vi "FlexMag - 24-03-2023.vi"() -> ()   [LabVIEW 2018] (continued)
            n4342 = Concatenate Strings("000000" ("string"), w7261) -> (w7255:string)
            n4343 = String Length(string=w7255) -> (length=w7257:i32)
            n4344 = Subtract(x=w7257, y=6) -> (x-y=w7259:i32)
            n4345 = String Subset(string=w7255, offset (0)=w7259) -> (substring=w7254:string)  [unwired: 1 out]
            n4346 = Concatenate Strings("#001R:" ("string"), w7254, "\r", "\n") -> (w7271:string)
            n4347 = VISA Write(VISA resource name=w7273, write buffer=w7271, error in (no error)=w7272) -> (VISA resource name out=w7246:refnum<visa-resource-name>, error out=w7245:errorcluster)  [unwired: 1 out]
            n4348 = stacked-sequence {
              tunnel: [w7279] -> w7253
              tunnel: w7246 -> [w7279]
              tunnel: [w7278] -> w7252
              tunnel: w7245 -> [w7278]
              frame #0 {
                n4349 = Wait (ms)(milliseconds to wait=u32 50) -> ()  [unwired: 1 out]
              }
            }
            n4350 = property class="Instr"(reference=w7253, error in=w7252) -> (reference out=w7249:refnum<visa-resource-name>, error out=w7251:errorcluster, "Serial Settings:Number of Bytes at Serial Port"=w7250:u32)
            n4351 = VISA Read(VISA resource name=w7249, byte count=w7250, error in (no error)=w7251) -> (VISA resource name out=w7248:refnum<visa-resource-name>, error out=w7247:errorcluster)  [unwired: 2 out]
            n4352 = local write "pcgv1 auto set position"(FALSE ("Pc_bv1_auto_set position")) -> ()
            n4353 = stacked-sequence {
              tunnel: [w7276] -> w7244
              tunnel: w7248 -> [w7276]
              tunnel: [w7275] -> w7243
              tunnel: w7247 -> [w7275]
              frame #0 {
                n4354 = Wait (ms)(milliseconds to wait=u32 50) -> ()  [unwired: 1 out]
              }
            }
          }
          frame 4 {
            n4355 = Multiply(x="pcgv1 set pressure value mbar", y=u16 750) -> (x*y=w7280:dbl)
            "pcgv1 setted pressure value torr" <- w7280
            n4356 = Multiply(x=w7280, y=10000.0) -> (x*y=w7301:dbl)
            n4357 = Number To Decimal String(number=w7301) -> (decimal integer string=w7295:string)  [unwired: 1 out]
            n4358 = Concatenate Strings("00000000" ("string"), w7295) -> (w7297:string)
            n4359 = String Length(string=w7297) -> (length=w7298:i32)
            n4360 = Subtract(x=w7298, y=8) -> (x-y=w7300:i32)
            n4361 = String Subset(string=w7297, offset (0)=w7300) -> (substring=w7294:string)  [unwired: 1 out]
            n4362 = Concatenate Strings("#001S:" ("string"), w7294, "\r", "\n") -> (w7302:string)
            n4363 = VISA Write(VISA resource name=w7309, write buffer=w7302, error in (no error)=w7308) -> (VISA resource name out=w7286:refnum<visa-resource-name>, error out=w7285:errorcluster)  [unwired: 1 out]
            n4364 = stacked-sequence {
              tunnel: [w7315] -> w7293
              tunnel: w7286 -> [w7315]
              tunnel: [w7314] -> w7292
              tunnel: w7285 -> [w7314]
              frame #0 {
                n4365 = Wait (ms)(milliseconds to wait=u32 50) -> ()  [unwired: 1 out]
              }
            }
            n4366 = property class="Instr"(reference=w7293, error in=w7292) -> (reference out=w7289:refnum<visa-resource-name>, error out=w7291:errorcluster, "Serial Settings:Number of Bytes at Serial Port"=w7290:u32)
            n4367 = VISA Read(VISA resource name=w7289, byte count=w7290, error in (no error)=w7291) -> (VISA resource name out=w7288:refnum<visa-resource-name>, error out=w7287:errorcluster)  [unwired: 2 out]
            n4368 = stacked-sequence {
              tunnel: [w7312] -> w7284
              tunnel: w7288 -> [w7312]
              tunnel: [w7311] -> w7283
              tunnel: w7287 -> [w7311]
              frame #0 {
                n4369 = Wait (ms)(milliseconds to wait=u32 50) -> ()  [unwired: 1 out]
              }
            }
            n4370 = local write "pcgv1 auto set pressure"(FALSE ("Pc_bv1_auto_set_pressure")) -> ()
          }
          frame 5 {
            n4371 = local write "Baratron1 auto set zero"(FALSE ("Pc_bv1_auto_baratron_set_zero")) -> ()
            n4372 = Concatenate Strings("#001Z:" ("string"), "\r", "\n") -> (w7329:string)
            n4373 = VISA Write(VISA resource name=w7333, write buffer=w7329, error in (no error)=w7332) -> (VISA resource name out=w7319:refnum<visa-resource-name>, error out=w7318:errorcluster)  [unwired: 1 out]
            n4374 = stacked-sequence {
              tunnel: [w7339] -> w7326
              tunnel: w7319 -> [w7339]
              tunnel: [w7338] -> w7325
              tunnel: w7318 -> [w7338]
              frame #0 {
                n4375 = Wait (ms)(milliseconds to wait=u32 50) -> ()  [unwired: 1 out]
              }
            }
            n4376 = property class="Instr"(reference=w7326, error in=w7325) -> (reference out=w7322:refnum<visa-resource-name>, error out=w7324:errorcluster, "Serial Settings:Number of Bytes at Serial Port"=w7323:u32)
            n4377 = VISA Read(VISA resource name=w7322, byte count=w7323, error in (no error)=w7324) -> (VISA resource name out=w7321:refnum<visa-resource-name>, error out=w7320:errorcluster)  [unwired: 2 out]
            n4378 = stacked-sequence {
              tunnel: [w7336] -> w7317
              tunnel: w7321 -> [w7336]
              tunnel: [w7335] -> w7316
              tunnel: w7320 -> [w7335]
              frame #0 {
                n4379 = Wait (ms)(milliseconds to wait=u32 50) -> ()  [unwired: 1 out]
              }
            }
          }
          frame 6 {
            n4380 = Concatenate Strings("#001L:" ("string"), "Learn value", "\r", "\n") -> (w7353:string)
            n4381 = VISA Write(VISA resource name=w7357, write buffer=w7353, error in (no error)=w7356) -> (VISA resource name out=w7343:refnum<visa-resource-name>, error out=w7342:errorcluster)  [unwired: 1 out]
            n4382 = stacked-sequence {
              tunnel: [w7363] -> w7350
              tunnel: w7343 -> [w7363]
              tunnel: [w7362] -> w7349
              tunnel: w7342 -> [w7362]
              frame #0 {
                n4383 = Wait (ms)(milliseconds to wait=u32 50) -> ()  [unwired: 1 out]
              }
            }
            n4384 = property class="Instr"(reference=w7350, error in=w7349) -> (reference out=w7346:refnum<visa-resource-name>, error out=w7348:errorcluster, "Serial Settings:Number of Bytes at Serial Port"=w7347:u32)
            n4385 = VISA Read(VISA resource name=w7346, byte count=w7347, error in (no error)=w7348) -> (VISA resource name out=w7345:refnum<visa-resource-name>, error out=w7344:errorcluster)  [unwired: 2 out]
            n4386 = stacked-sequence {
              tunnel: [w7360] -> w7341
              tunnel: w7345 -> [w7360]
              tunnel: [w7359] -> w7340
              tunnel: w7344 -> [w7359]
              frame #0 {
                n4387 = Wait (ms)(milliseconds to wait=u32 50) -> ()  [unwired: 1 out]
              }
            }
          }
        }
      }
      frame #1 {
        n4388 = Or(x="pcgv2 set position gui", y="pcgv2 auto set position") -> (x .or. y?=w7386:bool)
        n4389 = Or(x="pcgv2 set pressure gui", y="pcgv2 auto set pressure") -> (x .or. y?=w7385:bool)
        n4390 = Compound Arithmetic op=OR("pcgv2 open gui 2", "pcgv2 open gui 1", "pcgv2 open gui", "pcgv2 auto open") -> (w7371:bool)
        n4391 = Compound Arithmetic op=OR("pcgv2 close gui 2", "pcgv2 close gui 1", "pcgv2 auto close", "pcgv2 close gui") -> (w7370:bool)
        n4392 = Or(x="Baratron2 set zero gui", y="Baratron2 auto set zero") -> (x .or. y?=w7384:bool)
        n4393 = Build Array(FALSE, w7371, w7370, w7386, w7385, w7384) -> (w7388:bool[])
        n4394 = Boolean Array To Number(Boolean array=w7388) -> (number=w7390:u32)
        n4395 = Mantissa & Exponent(0:w7390) -> (2:w7389:dbl)  [unwired: 1 out]
        n4396 = case shown="0, Default" w7389 {
          tunnel: [w7394 w7463 w7486 w7509 w7549 w7583] -> w7368
          tunnel: [w7393 w7464 w7485 w7510 w7550 w7582] -> w7367
          tunnel: w7369 -> [w7392 w7473 w7497 w7521 w7561 w7594]
          tunnel: w7366 -> [w7391 w7472 w7496 w7520 w7560 w7593]
          frame 0, Default {
            n4397 = stacked-sequence {
              seq-local: [_ w7399 _ _ _] -> [_ _ _ w7436 _]
              seq-local: [_ w7398 _ _ _] -> [_ _ _ w7435 _]
              tunnel: [_ _ _ w7438 _] -> w7394
              tunnel: [_ _ _ w7437 _] -> w7393
              tunnel: w7392 -> [_ w7397 _ _ _]
              tunnel: w7391 -> [_ w7396 _ _ _]
              frame #0 {
                n4398 = Wait (ms)(milliseconds to wait=u32 50) -> ()  [unwired: 1 out]
              }
              frame #1 {
                n4399 = Concatenate Strings("#002A:" ("string"), "\r", "\n") -> (w7415:string)
                n4400 = VISA Write(VISA resource name=w7397, write buffer=w7415, error in (no error)=w7396) -> (VISA resource name out=w7413:refnum<visa-resource-name>, error out=w7412:errorcluster)  [unwired: 1 out]
                n4401 = stacked-sequence {
                  tunnel: [w7420] -> w7411
                  tunnel: w7413 -> [w7420]
                  tunnel: [w7419] -> w7410
                  tunnel: w7412 -> [w7419]
                  frame #0 {
                    n4402 = Wait (ms)(milliseconds to wait=u32 50) -> ()  [unwired: 1 out]
                  }
                }
                n4403 = property class="Instr"(reference=w7411, error in=w7410) -> (reference out=w7407:refnum<visa-resource-name>, error out=w7409:errorcluster, "Serial Settings:Number of Bytes at Serial Port"=w7408:u32)
                n4404 = VISA Read(VISA resource name=w7407, byte count=w7408, error in (no error)=w7409) -> (VISA resource name out=w7399:refnum<visa-resource-name>, read buffer=w7401:string, error out=w7398:errorcluster)  [unwired: 1 out]
                n4405 = Match Pattern(string=w7401, regular expression="#002A:") -> (after substring=w7405:string)  [unwired: 1 in, 3 out]
                n4406 = String Subset(string=w7405, offset (0)=0, length (rest)=3 ("length (rest)")) -> (substring=w7402:string)
                n4407 = Decimal String To Number(string=w7402) -> (number=→"pcgv2 position":i32)  [unwired: 2 in, 1 out]
              }
              frame #2 {
                n4408 = Wait (ms)(milliseconds to wait=u32 50) -> ()  [unwired: 1 out]
              }
              frame #3 {
                n4409 = Concatenate Strings("#002P:" ("string"), "\r", "\n") -> (w7452:string)
                n4410 = VISA Write(VISA resource name=w7436, write buffer=w7452, error in (no error)=w7435) -> (VISA resource name out=w7450:refnum<visa-resource-name>, error out=w7449:errorcluster)  [unwired: 1 out]
                n4411 = stacked-sequence {
                  tunnel: [w7459] -> w7448
                  tunnel: w7450 -> [w7459]
                  tunnel: [w7458] -> w7447
                  tunnel: w7449 -> [w7458]
                  frame #0 {
                    n4412 = Wait (ms)(milliseconds to wait=u32 50) -> ()  [unwired: 1 out]
                  }
                }
                n4413 = property class="Instr"(reference=w7448, error in=w7447) -> (reference out=w7444:refnum<visa-resource-name>, error out=w7446:errorcluster, "Serial Settings:Number of Bytes at Serial Port"=w7445:u32)
                n4414 = VISA Read(VISA resource name=w7444, byte count=w7445, error in (no error)=w7446) -> (VISA resource name out=w7438:refnum<visa-resource-name>, read buffer=w7439:string, error out=w7437:errorcluster)  [unwired: 1 out]
                n4415 = Match Pattern(string=w7439, regular expression="#002P:") -> (after substring=w7427:string)  [unwired: 1 in, 3 out]
                n4416 = String Subset(string=w7427, offset (0)=0, length (rest)=1 ("length (rest)")) -> (substring=w7430:string)
                n4417 = String Subset(string=w7427, offset (0)=2, length (rest)=4 ("length (rest)")) -> (substring=w7440:string)
                n4418 = Equal?(x=w7430, y="-") -> (x = y?=w7428:bool)
                n4419 = Decimal String To Number(string=w7440) -> (number=w7434:i32)  [unwired: 2 in, 1 out]
                n4420 = case shown="True" w7428 {
                  frame False {
                  }
                  frame True {
                    w7455 = u16 0 ("Ch2_baratron_pressure_mbar")
                    w7456 = 0 ("Pressure 2")
                    n4421 = local write "Pressure 2_gui"(w7456) -> ()
                    n4422 = local write "Pressure 2_gui 2"(w7456) -> ()
                    n4423 = local write "Pressure 2"(w7456) -> ()
                    n4424 = local write "Ch2_baratron_pressure_mbar 2"(w7455) -> ()
                    n4425 = local write "Ch2_baratron_pressure_mbar"(w7455) -> ()
                    n4426 = local write "Ch2_baratron_pressure_mbar 3"(w7455) -> ()
                  }
                }
                n4427 = Divide(x=w7434, y=100) -> (x/y=w7425:dbl)
                "Pressure 2" <- w7425
                "Pressure 2_gui" <- w7425
                "Pressure 2_gui 2" <- w7425
                n4428 = Multiply(x=w7425, y=0.00133) -> (x*y=w7424:dbl)
                "Ch2_baratron_pressure_mbar" <- w7424
                "Ch2_baratron_pressure_mbar 2" <- w7424
                "Ch2_baratron_pressure_mbar 3" <- w7424
                n4429 = Number To Exponential String(number=w7424, precision (6)=i16 3) -> (E-format string=→"CH2 CH BG":string)  [unwired: 2 in]
              }
              frame #4 {
                n4430 = Wait (ms)(milliseconds to wait=u32 50) -> ()  [unwired: 1 out]
              }
            }
          }
          frame 1 {
            n4431 = Concatenate Strings("#002O:" ("string"), "\r", "\n") -> (w7476:string)
            n4432 = VISA Write(VISA resource name=w7473, write buffer=w7476, error in (no error)=w7472) -> (VISA resource name out=w7461:refnum<visa-resource-name>, error out=w7462:errorcluster)  [unwired: 1 out]
            n4433 = stacked-sequence {
              tunnel: [w7484] -> w7471
              tunnel: w7461 -> [w7484]
              tunnel: [w7483] -> w7470
              tunnel: w7462 -> [w7483]
              frame #0 {
                n4434 = Wait (ms)(milliseconds to wait=u32 50) -> ()  [unwired: 1 out]
              }
            }
            n4435 = local write "pcgv2 auto open"(FALSE ("Pc_bv2_auto_open")) -> ()
            n4436 = property class="Instr"(reference=w7471, error in=w7470) -> (reference out=w7467:refnum<visa-resource-name>, error out=w7469:errorcluster, "Serial Settings:Number of Bytes at Serial Port"=w7468:u32)
            n4437 = VISA Read(VISA resource name=w7467, byte count=w7468, error in (no error)=w7469) -> (VISA resource name out=w7466:refnum<visa-resource-name>, error out=w7465:errorcluster)  [unwired: 2 out]
            n4438 = stacked-sequence {
              tunnel: [w7481] -> w7463
              tunnel: w7466 -> [w7481]
              tunnel: [w7480] -> w7464
              tunnel: w7465 -> [w7480]
              frame #0 {
                n4439 = Wait (ms)(milliseconds to wait=u32 50) -> ()  [unwired: 1 out]
              }
            }
          }
          frame 2 {
            n4440 = Concatenate Strings("#002C:" ("string"), "\r", "\n") -> (w7500:string)
            n4441 = VISA Write(VISA resource name=w7497, write buffer=w7500, error in (no error)=w7496) -> (VISA resource name out=w7488:refnum<visa-resource-name>, error out=w7487:errorcluster)  [unwired: 1 out]
            n4442 = local write "pcgv2 auto close"(FALSE ("Pc_bv2_auto_close")) -> ()
            n4443 = stacked-sequence {
              tunnel: [w7508] -> w7495
              tunnel: w7488 -> [w7508]
              tunnel: [w7507] -> w7494
              tunnel: w7487 -> [w7507]
              frame #0 {
                n4444 = Wait (ms)(milliseconds to wait=u32 50) -> ()  [unwired: 1 out]
              }
            }
            n4445 = property class="Instr"(reference=w7495, error in=w7494) -> (reference out=w7491:refnum<visa-resource-name>, error out=w7493:errorcluster, "Serial Settings:Number of Bytes at Serial Port"=w7492:u32)
            n4446 = VISA Read(VISA resource name=w7491, byte count=w7492, error in (no error)=w7493) -> (VISA resource name out=w7490:refnum<visa-resource-name>, error out=w7489:errorcluster)  [unwired: 2 out]
            n4447 = stacked-sequence {
              tunnel: [w7505] -> w7486
              tunnel: w7490 -> [w7505]
              tunnel: [w7504] -> w7485
              tunnel: w7489 -> [w7504]
              frame #0 {
                n4448 = Wait (ms)(milliseconds to wait=u32 50) -> ()  [unwired: 1 out]
              }
            }
          }
          frame 3 {
            n4449 = In Range and Coerce(upper limit=100.0, x="pcgv2 set position value", lower limit=0.0) -> (coerced(x)=w7523:dbl)  [unwired: 1 out]
            n4450 = Multiply(x=w7523, y=1000.0) -> (x*y=w7530:dbl)
            n4451 = Number To Decimal String(number=w7530) -> (decimal integer string=w7532:string)  [unwired: 1 out]
            n4452 = Concatenate Strings("000000" ("string"), w7532) -> (w7534:string)
            n4453 = String Length(string=w7534) -> (length=w7535:i32)
            n4454 = Subtract(x=w7535, y=6) -> (x-y=w7537:i32)
            n4455 = String Subset(string=w7534, offset (0)=w7537) -> (substring=w7527:string)  [unwired: 1 out]
            n4456 = Concatenate Strings("#002R:" ("string"), w7527, "\r", "\n") -> (w7539:string)
            n4457 = VISA Write(VISA resource name=w7521, write buffer=w7539, error in (no error)=w7520) -> (VISA resource name out=w7513:refnum<visa-resource-name>, error out=w7512:errorcluster)  [unwired: 1 out]
            n4458 = stacked-sequence {
              tunnel: [w7544] -> w7514
              tunnel: w7513 -> [w7544]
              tunnel: [w7543] -> w7511
              tunnel: w7512 -> [w7543]
              frame #0 {
                n4459 = Wait (ms)(milliseconds to wait=u32 50) -> ()  [unwired: 1 out]
              }
            }
            n4460 = property class="Instr"(reference=w7514, error in=w7511) -> (reference out=w7517:refnum<visa-resource-name>, error out=w7519:errorcluster, "Serial Settings:Number of Bytes at Serial Port"=w7518:u32)
            n4461 = VISA Read(VISA resource name=w7517, byte count=w7518, error in (no error)=w7519) -> (VISA resource name out=w7516:refnum<visa-resource-name>, error out=w7515:errorcluster)  [unwired: 2 out]
            n4462 = local write "pcgv2 auto set position"(FALSE ("Pc_bv2_auto_set position")) -> ()
            n4463 = stacked-sequence {
              tunnel: [w7542] -> w7509
              tunnel: w7516 -> [w7542]
              tunnel: [w7541] -> w7510
              tunnel: w7515 -> [w7541]
              frame #0 {
                n4464 = Wait (ms)(milliseconds to wait=u32 50) -> ()  [unwired: 1 out]
              }
            }
          }
          frame 4 {
            n4465 = Multiply(x="pcgv2 set pressure value mbar", y=u16 750) -> (x*y=w7546:dbl)
            "pcgv2 setted pressure value torr" <- w7546
            n4466 = Multiply(x=w7546, y=10000.0) -> (x*y=w7566:dbl)
            n4467 = Number To Decimal String(number=w7566) -> (decimal integer string=w7568:string)  [unwired: 1 out]
            n4468 = Concatenate Strings("00000000" ("string"), w7568) -> (w7570:string)
            n4469 = String Length(string=w7570) -> (length=w7571:i32)
            n4470 = Subtract(x=w7571, y=8) -> (x-y=w7573:i32)
            n4471 = String Subset(string=w7570, offset (0)=w7573) -> (substring=w7563:string)  [unwired: 1 out]
            n4472 = Concatenate Strings("#002S:" ("string"), w7563, "\r", "\n") -> (w7575:string)
            n4473 = VISA Write(VISA resource name=w7561, write buffer=w7575, error in (no error)=w7560) -> (VISA resource name out=w7552:refnum<visa-resource-name>, error out=w7551:errorcluster)  [unwired: 1 out]
            n4474 = stacked-sequence {
              tunnel: [w7580] -> w7554
              tunnel: w7552 -> [w7580]
              tunnel: [w7579] -> w7553
              tunnel: w7551 -> [w7579]
              frame #0 {
                n4475 = Wait (ms)(milliseconds to wait=u32 50) -> ()  [unwired: 1 out]
              }
            }
            n4476 = property class="Instr"(reference=w7554, error in=w7553) -> (reference out=w7557:refnum<visa-resource-name>, error out=w7559:errorcluster, "Serial Settings:Number of Bytes at Serial Port"=w7558:u32)
            n4477 = VISA Read(VISA resource name=w7557, byte count=w7558, error in (no error)=w7559) -> (VISA resource name out=w7556:refnum<visa-resource-name>, error out=w7555:errorcluster)  [unwired: 2 out]
            n4478 = local write "pcgv2 auto set pressure"(FALSE ("Pc_bv2_auto_set_pressure")) -> ()
            n4479 = stacked-sequence {
              tunnel: [w7578] -> w7549
              tunnel: w7556 -> [w7578]
              tunnel: [w7577] -> w7550
              tunnel: w7555 -> [w7577]
              frame #0 {
                n4480 = Wait (ms)(milliseconds to wait=u32 50) -> ()  [unwired: 1 out]
              }
            }
          }
          frame 5 {
            n4481 = Concatenate Strings("#002Z:" ("string"), "\r", "\n") -> (w7597:string)
            n4482 = VISA Write(VISA resource name=w7594, write buffer=w7597, error in (no error)=w7593) -> (VISA resource name out=w7585:refnum<visa-resource-name>, error out=w7584:errorcluster)  [unwired: 1 out]
            n4483 = stacked-sequence {
              tunnel: [w7604] -> w7587
              tunnel: w7585 -> [w7604]
              tunnel: [w7603] -> w7586
              tunnel: w7584 -> [w7603]
              frame #0 {
                n4484 = Wait (ms)(milliseconds to wait=u32 50) -> ()  [unwired: 1 out]
              }
            }
            n4485 = property class="Instr"(reference=w7587, error in=w7586) -> (reference out=w7590:refnum<visa-resource-name>, error out=w7592:errorcluster, "Serial Settings:Number of Bytes at Serial Port"=w7591:u32)
            n4486 = local write "Baratron2 auto set zero"(FALSE ("Pc_bv2_auto_baratron_set_zero")) -> ()
            n4487 = VISA Read(VISA resource name=w7590, byte count=w7591, error in (no error)=w7592) -> (VISA resource name out=w7589:refnum<visa-resource-name>, error out=w7588:errorcluster)  [unwired: 2 out]
            n4488 = stacked-sequence {
              tunnel: [w7602] -> w7583
              tunnel: w7589 -> [w7602]
              tunnel: [w7601] -> w7582
              tunnel: w7588 -> [w7601]
              frame #0 {
                n4489 = Wait (ms)(milliseconds to wait=u32 50) -> ()  [unwired: 1 out]
              }
            }
          }
        }
      }
      frame #2 {
        n4490 = Compound Arithmetic op=OR("pcgv3 open gui 2", "pcgv3 open gui 1", "pcgv3 open gui", "pcgv3 auto open") -> (w7616:bool)
        n4491 = Or(x="pcgv3 set pressure gui", y="pcgv3 auto set pressure") -> (x .or. y?=w7626:bool)
        n4492 = Compound Arithmetic op=OR("pcgv3 close gui 2", "pcgv3 close gui 1", "pcgv3 close gui", "pcgv3 auto close") -> (w7612:bool)
        n4493 = Or(x="pcgv3 set position", y="pcgv3 auto set position") -> (x .or. y?=w7627:bool)
        n4494 = Or(x="Baratron3 set zero gui", y="Baratron3 auto set zero") -> (x .or. y?=w7623:bool)
        n4495 = Build Array(FALSE, w7616, w7612, w7627, w7626, w7623) -> (w7630:bool[])
        n4496 = Boolean Array To Number(Boolean array=w7630) -> (number=w7632:u32)
        n4497 = Mantissa & Exponent(0:w7632) -> (2:w7631:dbl)  [unwired: 1 out]
        n4498 = case shown="0, Default" w7631 {
          tunnel: [w7636 w7703 w7728 w7752 w7792 w7825 w7849] -> w7610
          tunnel: [w7635 w7705 w7727 w7751 w7791 w7824 w7848] -> w7609
          tunnel: w7608 -> [w7634 w7715 w7739 w7763 w7803 w7836 w7860]
          tunnel: w7611 -> [w7633 w7714 w7738 w7762 w7802 w7835 w7859]
          frame 0, Default {
            n4499 = stacked-sequence {
              seq-local: [_ w7641 _ _ _] -> [_ _ _ w7679 _]
              seq-local: [_ w7640 _ _ _] -> [_ _ _ w7678 _]
              tunnel: [_ _ _ w7680 _] -> w7636
              tunnel: [_ _ _ w7672 _] -> w7635
              tunnel: w7634 -> [_ w7639 _ _ _]
              tunnel: w7633 -> [_ w7638 _ _ _]
              frame #0 {
                n4500 = Wait (ms)(milliseconds to wait=u32 50) -> ()  [unwired: 1 out]
              }
              frame #1 {
                n4501 = Concatenate Strings("#003A:" ("string"), "\r", "\n") -> (w7657:string)
                n4502 = VISA Write(VISA resource name=w7639, write buffer=w7657, error in (no error)=w7638) -> (VISA resource name out=w7655:refnum<visa-resource-name>, error out=w7654:errorcluster)  [unwired: 1 out]
                n4503 = stacked-sequence {
                  tunnel: [w7662] -> w7653
                  tunnel: w7655 -> [w7662]
                  tunnel: [w7661] -> w7652
                  tunnel: w7654 -> [w7661]
                  frame #0 {
                    n4504 = Wait (ms)(milliseconds to wait=u32 50) -> ()  [unwired: 1 out]
                  }
                }
                n4505 = property class="Instr"(reference=w7653, error in=w7652) -> (reference out=w7649:refnum<visa-resource-name>, error out=w7651:errorcluster, "Serial Settings:Number of Bytes at Serial Port"=w7650:u32)
                n4506 = VISA Read(VISA resource name=w7649, byte count=w7650, error in (no error)=w7651) -> (VISA resource name out=w7641:refnum<visa-resource-name>, read buffer=w7643:string, error out=w7640:errorcluster)  [unwired: 1 out]
                n4507 = Match Pattern(string=w7643, regular expression="#003A:") -> (after substring=w7647:string)  [unwired: 1 in, 3 out]
                n4508 = String Subset(string=w7647, offset (0)=0, length (rest)=3 ("length (rest)")) -> (substring=w7644:string)
                n4509 = Decimal String To Number(string=w7644) -> (number=→"pcgv3 position":i32)  [unwired: 2 in, 1 out]
              }
              frame #2 {
                n4510 = Wait (ms)(milliseconds to wait=u32 50) -> ()  [unwired: 1 out]
              }
              frame #3 {
                n4511 = Concatenate Strings("#003P:" ("string"), "\r", "\n") -> (w7694:string)
                n4512 = VISA Write(VISA resource name=w7679, write buffer=w7694, error in (no error)=w7678) -> (VISA resource name out=w7692:refnum<visa-resource-name>, error out=w7691:errorcluster)  [unwired: 1 out]
                n4513 = stacked-sequence {
                  tunnel: [w7701] -> w7690
                  tunnel: w7692 -> [w7701]
                  tunnel: [w7700] -> w7689
                  tunnel: w7691 -> [w7700]
                  frame #0 {
                    n4514 = Wait (ms)(milliseconds to wait=u32 50) -> ()  [unwired: 1 out]
                  }
                }
                n4515 = property class="Instr"(reference=w7690, error in=w7689) -> (reference out=w7686:refnum<visa-resource-name>, error out=w7688:errorcluster, "Serial Settings:Number of Bytes at Serial Port"=w7687:u32)
                n4516 = VISA Read(VISA resource name=w7686, byte count=w7687, error in (no error)=w7688) -> (VISA resource name out=w7680:refnum<visa-resource-name>, read buffer=w7681:string, error out=w7672:errorcluster)  [unwired: 1 out]
                n4517 = Match Pattern(string=w7681, regular expression="#003P:") -> (after substring=w7673:string)  [unwired: 1 in, 3 out]
                n4518 = String Subset(string=w7673, offset (0)=2, length (rest)=4 ("length (rest)")) -> (substring=w7682:string)
                n4519 = String Subset(string=w7673, offset (0)=0, length (rest)=1 ("length (rest)")) -> (substring=w7671:string)
                n4520 = Equal?(x=w7671, y="-" ("substring")) -> (x = y?=w7669:bool)
                n4521 = Decimal String To Number(string=w7682) -> (number=w7677:i32)  [unwired: 2 in, 1 out]
                n4522 = case shown="True" w7669 {
                  frame False {
                  }
                  frame True {
                    w7697 = u16 0 ("Ch3_baratron_pressure_mbar")
                    w7698 = 0 ("Pressure_ch3")
                    n4523 = local write "Pressure_ch3"(w7698) -> ()
                    n4524 = local write "Pressure ch3_gui"(w7698) -> ()
                    n4525 = local write "Pressure ch3_gui2"(w7698) -> ()
                    n4526 = local write "Ch3_baratron_pressure_mbar"(w7697) -> ()
                    n4527 = local write "Ch3_baratron_pressure_mbar 2"(w7697) -> ()
                    n4528 = local write "Ch3_baratron_pressure_mbar 3"(w7697) -> ()
                  }
                }
                n4529 = Divide(x=w7677, y=100) -> (x/y=w7667:dbl)
                "Pressure_ch3" <- w7667
                "Pressure ch3_gui" <- w7667
                "Pressure ch3_gui2" <- w7667
                n4530 = Multiply(x=w7667, y=0.00133) -> (x*y=w7665:dbl)
                "Ch3_baratron_pressure_mbar" <- w7665
                "Ch3_baratron_pressure_mbar 2" <- w7665
                "Ch3_baratron_pressure_mbar 3" <- w7665
                n4531 = Number To Exponential String(number=w7665, precision (6)=i16 3) -> (E-format string=→"CH3 CH BG":string)  [unwired: 2 in]
              }
              frame #4 {
                n4532 = Wait (ms)(milliseconds to wait=u32 50) -> ()  [unwired: 1 out]
              }
            }
          }
          frame 1 {
            n4533 = Concatenate Strings("#003O:" ("string"), "\r", "\n") -> (w7718:string)
            n4534 = VISA Write(VISA resource name=w7715, write buffer=w7718, error in (no error)=w7714) -> (VISA resource name out=w7704:refnum<visa-resource-name>, error out=w7706:errorcluster)  [unwired: 1 out]
            n4535 = stacked-sequence {
              tunnel: [w7726] -> w7713
              tunnel: w7704 -> [w7726]
              tunnel: [w7725] -> w7712
              tunnel: w7706 -> [w7725]
              frame #0 {
                n4536 = Wait (ms)(milliseconds to wait=u32 50) -> ()  [unwired: 1 out]
              }
            }
            n4537 = property class="Instr"(reference=w7713, error in=w7712) -> (reference out=w7709:refnum<visa-resource-name>, error out=w7711:errorcluster, "Serial Settings:Number of Bytes at Serial Port"=w7710:u32)
            n4538 = local write "pcgv3 auto open"(FALSE ("Pc_bv3_auto_open")) -> ()
            n4539 = VISA Read(VISA resource name=w7709, byte count=w7710, error in (no error)=w7711) -> (VISA resource name out=w7708:refnum<visa-resource-name>, error out=w7707:errorcluster)  [unwired: 2 out]
            n4540 = stacked-sequence {
              tunnel: [w7723] -> w7703
              tunnel: w7708 -> [w7723]
              tunnel: [w7722] -> w7705
              tunnel: w7707 -> [w7722]
              frame #0 {
                n4541 = Wait (ms)(milliseconds to wait=u32 50) -> ()  [unwired: 1 out]
              }
            }
          }
          frame 2 {
            n4542 = Concatenate Strings("#003C:" ("string"), "\r", "\n") -> (w7742:string)
            n4543 = VISA Write(VISA resource name=w7739, write buffer=w7742, error in (no error)=w7738) -> (VISA resource name out=w7730:refnum<visa-resource-name>, error out=w7729:errorcluster)  [unwired: 1 out]
            n4544 = stacked-sequence {
              tunnel: [w7750] -> w7737
              tunnel: w7730 -> [w7750]
              tunnel: [w7749] -> w7736
              tunnel: w7729 -> [w7749]
              frame #0 {
                n4545 = Wait (ms)(milliseconds to wait=u32 50) -> ()  [unwired: 1 out]
              }
            }
            n4546 = local write "pcgv3 auto close"(FALSE ("Pc_bv3_auto_close")) -> ()
            n4547 = property class="Instr"(reference=w7737, error in=w7736) -> (reference out=w7733:refnum<visa-resource-name>, error out=w7735:errorcluster, "Serial Settings:Number of Bytes at Serial Port"=w7734:u32)
            n4548 = VISA Read(VISA resource name=w7733, byte count=w7734, error in (no error)=w7735) -> (VISA resource name out=w7732:refnum<visa-resource-name>, error out=w7731:errorcluster)  [unwired: 2 out]
            n4549 = stacked-sequence {
              tunnel: [w7747] -> w7728
              tunnel: w7732 -> [w7747]
              tunnel: [w7746] -> w7727
              tunnel: w7731 -> [w7746]
              frame #0 {
                n4550 = Wait (ms)(milliseconds to wait=u32 50) -> ()  [unwired: 1 out]
              }
            }
          }
          frame 3 {
            n4551 = In Range and Coerce(upper limit=100.0, x="pcgv3 set position value", lower limit=0.0) -> (coerced(x)=w7768:dbl)  [unwired: 1 out]
            n4552 = Multiply(x=w7768, y=1000.0) -> (x*y=w7772:dbl)
            n4553 = Number To Decimal String(number=w7772) -> (decimal integer string=w7774:string)  [unwired: 1 out]
            n4554 = Concatenate Strings("000000" ("string"), w7774) -> (w7776:string)
            n4555 = String Length(string=w7776) -> (length=w7777:i32)
            n4556 = Subtract(x=w7777, y=6) -> (x-y=w7779:i32)
            n4557 = String Subset(string=w7776, offset (0)=w7779) -> (substring=w7769:string)  [unwired: 1 out]
            n4558 = Concatenate Strings("#003R:" ("string"), w7769, "\r", "\n") -> (w7781:string)
            n4559 = VISA Write(VISA resource name=w7763, write buffer=w7781, error in (no error)=w7762) -> (VISA resource name out=w7756:refnum<visa-resource-name>, error out=w7754:errorcluster)  [unwired: 1 out]
            n4560 = stacked-sequence {
              tunnel: [w7786] -> w7755
              tunnel: w7756 -> [w7786]
              tunnel: w7754 -> [w7785]
              tunnel: [w7785] -> w7753
              frame #0 {
                n4561 = Wait (ms)(milliseconds to wait=u32 50) -> ()  [unwired: 1 out]
              }
            }
            n4562 = property class="Instr"(reference=w7755, error in=w7753) -> (reference out=w7759:refnum<visa-resource-name>, error out=w7761:errorcluster, "Serial Settings:Number of Bytes at Serial Port"=w7760:u32)
            n4563 = VISA Read(VISA resource name=w7759, byte count=w7760, error in (no error)=w7761) -> (VISA resource name out=w7758:refnum<visa-resource-name>, error out=w7757:errorcluster)  [unwired: 2 out]
            n4564 = local write "pcgv3 auto set position"(FALSE ("Pc_bv3_auto_set position")) -> ()
            n4565 = stacked-sequence {
              tunnel: [w7784] -> w7752
              tunnel: w7758 -> [w7784]
              tunnel: [w7783] -> w7751
              tunnel: w7757 -> [w7783]
              frame #0 {
                n4566 = Wait (ms)(milliseconds to wait=u32 50) -> ()  [unwired: 1 out]
              }
            }
          }
          frame 4 {
            n4567 = Multiply(x="pcgv3 set pressure value mbar", y=u16 750) -> (x*y=w7789:dbl)
            "pcgv3 setted pressure value torr" <- w7789
            n4568 = Multiply(x=w7789, y=10000.0) -> (x*y=w7808:dbl)
            n4569 = Number To Decimal String(number=w7808) -> (decimal integer string=w7810:string)  [unwired: 1 out]
            n4570 = Concatenate Strings("00000000" ("string"), w7810) -> (w7812:string)
            n4571 = String Length(string=w7812) -> (length=w7813:i32)
            n4572 = Subtract(x=w7813, y=8) -> (x-y=w7815:i32)
            n4573 = String Subset(string=w7812, offset (0)=w7815) -> (substring=w7805:string)  [unwired: 1 out]
            n4574 = Concatenate Strings("#003S:" ("string"), w7805, "\r", "\n") -> (w7817:string)
            n4575 = VISA Write(VISA resource name=w7803, write buffer=w7817, error in (no error)=w7802) -> (VISA resource name out=w7795:refnum<visa-resource-name>, error out=w7793:errorcluster)  [unwired: 1 out]
            n4576 = stacked-sequence {
              tunnel: [w7822] -> w7796
              tunnel: w7795 -> [w7822]
              tunnel: [w7821] -> w7794
              tunnel: w7793 -> [w7821]
              frame #0 {
                n4577 = Wait (ms)(milliseconds to wait=u32 50) -> ()  [unwired: 1 out]
              }
            }
            n4578 = property class="Instr"(reference=w7796, error in=w7794) -> (reference out=w7799:refnum<visa-resource-name>, error out=w7801:errorcluster, "Serial Settings:Number of Bytes at Serial Port"=w7800:u32)
            n4579 = local write "pcgv3 auto set pressure"(FALSE ("Pc_bv3_auto_set_pressure")) -> ()
            n4580 = VISA Read(VISA resource name=w7799, byte count=w7800, error in (no error)=w7801) -> (VISA resource name out=w7798:refnum<visa-resource-name>, error out=w7797:errorcluster)  [unwired: 2 out]
            n4581 = stacked-sequence {
              tunnel: [w7820] -> w7792
              tunnel: w7798 -> [w7820]
              tunnel: [w7819] -> w7791
              tunnel: w7797 -> [w7819]
              frame #0 {
                n4582 = Wait (ms)(milliseconds to wait=u32 50) -> ()  [unwired: 1 out]
              }
            }
          }
          frame 5 {
            n4583 = Concatenate Strings("#003Z:" ("string"), "\r", "\n") -> (w7839:string)
            n4584 = VISA Write(VISA resource name=w7836, write buffer=w7839, error in (no error)=w7835) -> (VISA resource name out=w7828:refnum<visa-resource-name>, error out=w7826:errorcluster)  [unwired: 1 out]
            n4585 = stacked-sequence {
              tunnel: [w7846] -> w7829
              tunnel: w7828 -> [w7846]
              tunnel: [w7845] -> w7827
              tunnel: w7826 -> [w7845]
              frame #0 {
                n4586 = Wait (ms)(milliseconds to wait=u32 50) -> ()  [unwired: 1 out]
              }
            }
            n4587 = local write "Baratron3 set zero gui"(FALSE ("Pc_bv3_auto_baratron_set_zero")) -> ()
            n4588 = property class="Instr"(reference=w7829, error in=w7827) -> (reference out=w7832:refnum<visa-resource-name>, error out=w7834:errorcluster, "Serial Settings:Number of Bytes at Serial Port"=w7833:u32)
            n4589 = VISA Read(VISA resource name=w7832, byte count=w7833, error in (no error)=w7834) -> (VISA resource name out=w7831:refnum<visa-resource-name>, error out=w7830:errorcluster)  [unwired: 2 out]
            n4590 = stacked-sequence {
              tunnel: [w7844] -> w7825
              tunnel: w7831 -> [w7844]
              tunnel: [w7843] -> w7824
              tunnel: w7830 -> [w7843]
              frame #0 {
                n4591 = Wait (ms)(milliseconds to wait=u32 50) -> ()  [unwired: 1 out]
              }
            }
          }
          frame 6 {
            n4592 = Concatenate Strings("#003s:" ("string"), "string", "\r", "\n") -> (w7865:string)
            n4593 = VISA Write(VISA resource name=w7860, write buffer=w7865, error in (no error)=w7859) -> (VISA resource name out=w7852:refnum<visa-resource-name>, error out=w7850:errorcluster)  [unwired: 1 out]
            n4594 = stacked-sequence {
              tunnel: [w7870] -> w7853
              tunnel: w7852 -> [w7870]
              tunnel: [w7869] -> w7851
              tunnel: w7850 -> [w7869]
              frame #0 {
                n4595 = Wait (ms)(milliseconds to wait=u32 50) -> ()  [unwired: 1 out]
              }
            }
            n4596 = property class="Instr"(reference=w7853, error in=w7851) -> (reference out=w7856:refnum<visa-resource-name>, error out=w7858:errorcluster, "Serial Settings:Number of Bytes at Serial Port"=w7857:u32)
            n4597 = VISA Read(VISA resource name=w7856, byte count=w7857, error in (no error)=w7858) -> (VISA resource name out=w7855:refnum<visa-resource-name>, error out=w7854:errorcluster)  [unwired: 2 out]
            n4598 = stacked-sequence {
              tunnel: [w7868] -> w7849
              tunnel: w7855 -> [w7868]
              tunnel: [w7867] -> w7848
              tunnel: w7854 -> [w7867]
              frame #0 {
                n4599 = Wait (ms)(milliseconds to wait=u32 50) -> ()  [unwired: 1 out]
              }
            }
          }
        }
      }
      frame #3 {
        n4600 = Compound Arithmetic op=OR("pcgv4 open gui 1", "pcgv4 open gui", "pcgv4 auto open", "pcgv4 open gui 2") -> (w7878:bool)
        n4601 = Or(x="pcgv4 set position gui", y="pcgv4 auto set position") -> (x .or. y?=w7889:bool)
        n4602 = Or(x="pcgv4 set pressure", y="pcgv4 auto set pressure") -> (x .or. y?=w7888:bool)
        n4603 = Or(x="Baratron4 auto set zero", y="Baratron4 set zero gui") -> (x .or. y?=w7887:bool)
        n4604 = Compound Arithmetic op=OR("pcgv4 close gui 1", "pcgv4 close gui", "pcgv4 auto close", "pcgv4 close gui 2") -> (w7879:bool)
        n4605 = Build Array(FALSE, w7878, w7879, w7889, w7888, w7887) -> (w7886:bool[])
        n4606 = Boolean Array To Number(Boolean array=w7886) -> (number=w7898:u32)
        n4607 = Mantissa & Exponent(0:w7898) -> (2:w7897:dbl)  [unwired: 1 out]
        n4608 = case shown="0, Default" w7897 {
          tunnel: [w7902 w7971 w7995 w8018 w8059 w8092] -> w7877
          tunnel: [w7901 w7970 w7994 w8019 w8058 w8091] -> w7876
          tunnel: w7875 -> [w7900 w7982 w8006 w8030 w8070 w8103]
          tunnel: w7874 -> [w7899 w7981 w8005 w8029 w8069 w8102]
          frame 0, Default {
            n4609 = stacked-sequence {
              seq-local: [_ w7907 _ _ _] -> [_ _ _ w7946 _]
              seq-local: [_ w7906 _ _ _] -> [_ _ _ w7943 _]
              tunnel: [_ _ _ w7948 _] -> w7902
              tunnel: [_ _ _ w7947 _] -> w7901
              tunnel: w7900 -> [_ w7905 _ _ _]
              tunnel: w7899 -> [_ w7904 _ _ _]
              frame #0 {
                n4610 = Wait (ms)(milliseconds to wait=u32 50) -> ()  [unwired: 1 out]
              }
              frame #1 {
                n4611 = Concatenate Strings("#004A:" ("string"), "\r", "\n") -> (w7923:string)
                n4612 = VISA Write(VISA resource name=w7905, write buffer=w7923, error in (no error)=w7904) -> (VISA resource name out=w7921:refnum<visa-resource-name>, error out=w7920:errorcluster)  [unwired: 1 out]
                n4613 = stacked-sequence {
                  tunnel: [w7928] -> w7919
                  tunnel: w7921 -> [w7928]
                  tunnel: [w7927] -> w7918
                  tunnel: w7920 -> [w7927]
                  frame #0 {
                    n4614 = Wait (ms)(milliseconds to wait=u32 50) -> ()  [unwired: 1 out]
                  }
                }
                n4615 = property class="Instr"(reference=w7919, error in=w7918) -> (reference out=w7915:refnum<visa-resource-name>, error out=w7917:errorcluster, "Serial Settings:Number of Bytes at Serial Port"=w7916:u32)
                n4616 = VISA Read(VISA resource name=w7915, byte count=w7916, error in (no error)=w7917) -> (VISA resource name out=w7907:refnum<visa-resource-name>, read buffer=w7909:string, error out=w7906:errorcluster)  [unwired: 1 out]
                n4617 = Match Pattern(string=w7909, regular expression="#004A:") -> (after substring=w7913:string)  [unwired: 1 in, 3 out]
                n4618 = String Subset(string=w7913, offset (0)=0, length (rest)=3 ("length (rest)")) -> (substring=w7910:string)
                n4619 = Decimal String To Number(string=w7910) -> (number=→"pcgv4 position":i32)  [unwired: 2 in, 1 out]
              }
              frame #2 {
                n4620 = Wait (ms)(milliseconds to wait=u32 50) -> ()  [unwired: 1 out]
              }
              frame #3 {
                n4621 = Concatenate Strings("#004P:" ("string"), "\r", "\n") -> (w7962:string)
                n4622 = VISA Write(VISA resource name=w7946, write buffer=w7962, error in (no error)=w7943) -> (VISA resource name out=w7960:refnum<visa-resource-name>, error out=w7959:errorcluster)  [unwired: 1 out]
                n4623 = stacked-sequence {
                  tunnel: [w7968] -> w7958
                  tunnel: w7960 -> [w7968]
                  tunnel: [w7967] -> w7957
                  tunnel: w7959 -> [w7967]
                  frame #0 {
                    n4624 = Wait (ms)(milliseconds to wait=u32 50) -> ()  [unwired: 1 out]
                  }
                }
                n4625 = property class="Instr"(reference=w7958, error in=w7957) -> (reference out=w7954:refnum<visa-resource-name>, error out=w7956:errorcluster, "Serial Settings:Number of Bytes at Serial Port"=w7955:u32)
                n4626 = VISA Read(VISA resource name=w7954, byte count=w7955, error in (no error)=w7956) -> (VISA resource name out=w7948:refnum<visa-resource-name>, read buffer=w7949:string, error out=w7947:errorcluster)  [unwired: 1 out]
                n4627 = Match Pattern(string=w7949, regular expression="#004P:") -> (after substring=w7937:string)  [unwired: 1 in, 3 out]
                n4628 = String Subset(string=w7937, offset (0)=0, length (rest)=1 ("length (rest)")) -> (substring=w7940:string)
                n4629 = String Subset(string=w7937, offset (0)=2, length (rest)=4 ("length (rest)")) -> (substring=w7950:string)
                n4630 = Equal?(x=w7940, y="-") -> (x = y?=w7938:bool)
                n4631 = Decimal String To Number(string=w7950) -> (number=w7945:i32)  [unwired: 2 in, 1 out]
                n4632 = case shown="True" w7938 {
                  frame False {
                  }
                  frame True {
                    w7965 = 0 ("Pressure 4")
                    n4633 = local write "Pressure 4"(w7965) -> ()
                    n4634 = local write "Pressurech4_gui"(w7965) -> ()
                    n4635 = local write "Pressurech4_gui 2"(w7965) -> ()
                    n4636 = local write "Ch4_baratron_pressure_mbar 2"(w7965) -> ()
                    n4637 = local write "Ch4_baratron_pressure_mbar"(w7965) -> ()
                    n4638 = local write "Ch4_baratron_pressure_mbar 3"(w7965) -> ()
                  }
                }
                n4639 = Divide(x=w7945, y=100) -> (x/y=w7935:dbl)
                "Pressure 4" <- w7935
                "Pressurech4_gui" <- w7935
                "Pressurech4_gui 2" <- w7935
                n4640 = Multiply(x=w7935, y=1.33) -> (x*y=w7934:dbl)
                n4641 = Divide(x=w7934, y=1000.0) -> (x/y=w7930:dbl)
                "Ch4_baratron_pressure_mbar" <- w7930
                "Ch4_baratron_pressure_mbar 2" <- w7930
                "Ch4_baratron_pressure_mbar 3" <- w7930
                n4642 = Number To Exponential String(number=w7930, precision (6)=i16 3) -> (E-format string=→"CH4 CH BG":string)  [unwired: 2 in]
              }
              frame #4 {
                n4643 = Wait (ms)(milliseconds to wait=u32 50) -> ()  [unwired: 1 out]
              }
            }
          }
          frame 1 {
            n4644 = Concatenate Strings("#004O:" ("string"), "\r", "\n") -> (w7985:string)
            n4645 = VISA Write(VISA resource name=w7982, write buffer=w7985, error in (no error)=w7981) -> (VISA resource name out=w7974:refnum<visa-resource-name>, error out=w7972:errorcluster)  [unwired: 1 out]
            n4646 = stacked-sequence {
              tunnel: [w7992] -> w7975
              tunnel: w7974 -> [w7992]
              tunnel: [w7991] -> w7973
              tunnel: w7972 -> [w7991]
              frame #0 {
                n4647 = Wait (ms)(milliseconds to wait=u32 50) -> ()  [unwired: 1 out]
              }
            }
            n4648 = local write "pcgv4 auto open"(FALSE ("Pc_bv4_auto_open")) -> ()
            n4649 = property class="Instr"(reference=w7975, error in=w7973) -> (reference out=w7978:refnum<visa-resource-name>, error out=w7980:errorcluster, "Serial Settings:Number of Bytes at Serial Port"=w7979:u32)
            n4650 = VISA Read(VISA resource name=w7978, byte count=w7979, error in (no error)=w7980) -> (VISA resource name out=w7977:refnum<visa-resource-name>, error out=w7976:errorcluster)  [unwired: 2 out]
            n4651 = stacked-sequence {
              tunnel: [w7990] -> w7971
              tunnel: w7977 -> [w7990]
              tunnel: [w7989] -> w7970
              tunnel: w7976 -> [w7989]
              frame #0 {
                n4652 = Wait (ms)(milliseconds to wait=u32 50) -> ()  [unwired: 1 out]
              }
            }
          }
          frame 2 {
            n4653 = Concatenate Strings("#004C:" ("string"), "\r", "\n") -> (w8009:string)
            n4654 = VISA Write(VISA resource name=w8006, write buffer=w8009, error in (no error)=w8005) -> (VISA resource name out=w7997:refnum<visa-resource-name>, error out=w7996:errorcluster)  [unwired: 1 out]
            n4655 = local write "pcgv4 auto close"(FALSE ("Pc_bv4_auto_close")) -> ()
            n4656 = stacked-sequence {
              tunnel: [w8016] -> w7999
              tunnel: w7997 -> [w8016]
              tunnel: [w8015] -> w7998
              tunnel: w7996 -> [w8015]
              frame #0 {
                n4657 = Wait (ms)(milliseconds to wait=u32 50) -> ()  [unwired: 1 out]
              }
            }
            n4658 = property class="Instr"(reference=w7999, error in=w7998) -> (reference out=w8002:refnum<visa-resource-name>, error out=w8004:errorcluster, "Serial Settings:Number of Bytes at Serial Port"=w8003:u32)
            n4659 = VISA Read(VISA resource name=w8002, byte count=w8003, error in (no error)=w8004) -> (VISA resource name out=w8001:refnum<visa-resource-name>, error out=w8000:errorcluster)  [unwired: 2 out]
            n4660 = stacked-sequence {
              tunnel: [w8014] -> w7995
              tunnel: w8001 -> [w8014]
              tunnel: [w8013] -> w7994
              tunnel: w8000 -> [w8013]
              frame #0 {
                n4661 = Wait (ms)(milliseconds to wait=u32 50) -> ()  [unwired: 1 out]
              }
            }
          }
          frame 3 {
            n4662 = In Range and Coerce(upper limit=100.0, x="pcgv4 set position value", lower limit=0.0) -> (coerced(x)=w8033:dbl)  [unwired: 1 out]
            n4663 = Multiply(x=w8033, y=1000.0) -> (x*y=w8040:dbl)
            n4664 = Number To Decimal String(number=w8040) -> (decimal integer string=w8041:string)  [unwired: 1 out]
            n4665 = Concatenate Strings("000000" ("string"), w8041) -> (w8043:string)
            n4666 = String Length(string=w8043) -> (length=w8044:i32)
            n4667 = Subtract(x=w8044, y=6) -> (x-y=w8046:i32)
            n4668 = String Subset(string=w8043, offset (0)=w8046) -> (substring=w8037:string)  [unwired: 1 out]
            n4669 = Concatenate Strings("#004R:" ("string"), w8037, "\r", "\n") -> (w8048:string)
            n4670 = VISA Write(VISA resource name=w8030, write buffer=w8048, error in (no error)=w8029) -> (VISA resource name out=w8021:refnum<visa-resource-name>, error out=w8020:errorcluster)  [unwired: 1 out]
            n4671 = stacked-sequence {
              tunnel: [w8053] -> w8023
              tunnel: w8021 -> [w8053]
              tunnel: [w8052] -> w8022
              tunnel: w8020 -> [w8052]
              frame #0 {
                n4672 = Wait (ms)(milliseconds to wait=u32 50) -> ()  [unwired: 1 out]
              }
            }
            n4673 = property class="Instr"(reference=w8023, error in=w8022) -> (reference out=w8026:refnum<visa-resource-name>, error out=w8028:errorcluster, "Serial Settings:Number of Bytes at Serial Port"=w8027:u32)
            n4674 = local write "pcgv4 auto set position"(FALSE ("Pc_bv4_auto_set position")) -> ()
            n4675 = VISA Read(VISA resource name=w8026, byte count=w8027, error in (no error)=w8028) -> (VISA resource name out=w8025:refnum<visa-resource-name>, error out=w8024:errorcluster)  [unwired: 2 out]
            n4676 = stacked-sequence {
              tunnel: [w8051] -> w8018
              tunnel: w8025 -> [w8051]
              tunnel: [w8050] -> w8019
              tunnel: w8024 -> [w8050]
              frame #0 {
                n4677 = Wait (ms)(milliseconds to wait=u32 50) -> ()  [unwired: 1 out]
              }
            }
          }
          frame 4 {
            n4678 = Multiply(x="pcgv4 set pressure value mbar", y=u16 750) -> (x*y=w8055:dbl)
            "pcgv4 setted pressure value torr" <- w8055
            n4679 = Multiply(x=w8055, y=10000.0) -> (x*y=w8075:dbl)
            n4680 = Number To Decimal String(number=w8075) -> (decimal integer string=w8077:string)  [unwired: 1 out]
            n4681 = Concatenate Strings("00000000" ("string"), w8077) -> (w8079:string)
            n4682 = String Length(string=w8079) -> (length=w8080:i32)
            n4683 = Subtract(x=w8080, y=8) -> (x-y=w8082:i32)
            n4684 = String Subset(string=w8079, offset (0)=w8082) -> (substring=w8072:string)  [unwired: 1 out]
            n4685 = Concatenate Strings("#004S:" ("string"), w8072, "\r", "\n") -> (w8084:string)
            n4686 = VISA Write(VISA resource name=w8070, write buffer=w8084, error in (no error)=w8069) -> (VISA resource name out=w8061:refnum<visa-resource-name>, error out=w8060:errorcluster)  [unwired: 1 out]
            n4687 = stacked-sequence {
              tunnel: [w8089] -> w8063
              tunnel: w8061 -> [w8089]
              tunnel: [w8088] -> w8062
              tunnel: w8060 -> [w8088]
              frame #0 {
                n4688 = Wait (ms)(milliseconds to wait=u32 50) -> ()  [unwired: 1 out]
              }
            }
            n4689 = property class="Instr"(reference=w8063, error in=w8062) -> (reference out=w8066:refnum<visa-resource-name>, error out=w8068:errorcluster, "Serial Settings:Number of Bytes at Serial Port"=w8067:u32)
            n4690 = local write "pcgv4 auto set pressure"(FALSE ("Pc_bv4_auto_set_pressure")) -> ()
            n4691 = VISA Read(VISA resource name=w8066, byte count=w8067, error in (no error)=w8068) -> (VISA resource name out=w8065:refnum<visa-resource-name>, error out=w8064:errorcluster)  [unwired: 2 out]
            n4692 = stacked-sequence {
              tunnel: [w8087] -> w8059
              tunnel: w8065 -> [w8087]
              tunnel: [w8086] -> w8058
              tunnel: w8064 -> [w8086]
              frame #0 {
                n4693 = Wait (ms)(milliseconds to wait=u32 50) -> ()  [unwired: 1 out]
              }
            }
          }
          frame 5 {
            n4694 = Concatenate Strings("#004Z:" ("string"), "\r", "\n") -> (w8106:string)
            n4695 = VISA Write(VISA resource name=w8103, write buffer=w8106, error in (no error)=w8102) -> (VISA resource name out=w8093:refnum<visa-resource-name>, error out=w8094:errorcluster)  [unwired: 1 out]
            n4696 = stacked-sequence {
              tunnel: [w8113] -> w8096
              tunnel: w8093 -> [w8113]
              tunnel: [w8112] -> w8095
              tunnel: w8094 -> [w8112]
              frame #0 {
                n4697 = Wait (ms)(milliseconds to wait=u32 50) -> ()  [unwired: 1 out]
              }
            }
            n4698 = local write "Baratron4 auto set zero"(FALSE ("Pc_bv4_auto_baratron_set_zero")) -> ()
            n4699 = property class="Instr"(reference=w8096, error in=w8095) -> (reference out=w8099:refnum<visa-resource-name>, error out=w8101:errorcluster, "Serial Settings:Number of Bytes at Serial Port"=w8100:u32)
            n4700 = VISA Read(VISA resource name=w8099, byte count=w8100, error in (no error)=w8101) -> (VISA resource name out=w8098:refnum<visa-resource-name>, error out=w8097:errorcluster)  [unwired: 2 out]
            n4701 = stacked-sequence {
              tunnel: [w8111] -> w8092
              tunnel: w8098 -> [w8111]
              tunnel: [w8110] -> w8091
              tunnel: w8097 -> [w8110]
              frame #0 {
                n4702 = Wait (ms)(milliseconds to wait=u32 50) -> ()  [unwired: 1 out]
              }
            }
          }
        }
      }
    }
    n4703 = Wait Until Next ms Multiple(millisecond multiple=u32 300) -> ()  [unwired: 1 out]
  }
  n4704 = while {
    tunnel: w94 -> [w8118]
    tunnel: w93 -> [w8117]
    tunnel: [w8116] -> w92
    tunnel: [w8115] -> w91
    stop <- FALSE stop-if-true
    n4705 = Wait Until Next ms Multiple(millisecond multiple=u32 300) -> ()  [unwired: 1 out]
    n4706 = stacked-sequence {
      seq-local: [w8125 _ _ _] -> [_ w8531 _ w9361]
      seq-local: [w8145 _ _ _] -> [_ w8549 _ w9362]
      seq-local: [_ w8527 _ _] -> [_ _ w8934 _]
      seq-local: [_ w8526 _ _] -> [_ _ w8933 _]
      seq-local: [_ _ w8932 _] -> [_ _ _ _]
      seq-local: [_ _ w8931 _] -> [_ _ _ _]
      tunnel: w8118 -> [w8123 _ _ _]
      tunnel: w8117 -> [w8122 _ _ _]
      tunnel: [_ _ _ w9360] -> w8116
      tunnel: [_ _ _ w9359] -> w8115
      frame #0 {
        n4707 = Or(x="Tp1 set speed gui", y="Tp1 auto set speed") -> (x .or. y?=w8141:bool)
        n4708 = Compound Arithmetic op=OR("Tp1 start gui", "Tp1 start gui 1", "Tp1 auto start") -> (w8124:bool)
        n4709 = Compound Arithmetic op=OR("Tp1 stop gui", "Tp1 stop gui 1", "Tp1 auto stop") -> (w8126:bool)
        n4710 = Or(x="Tp1 low speed gui", y="Tp1 auto low speed") -> (x .or. y?=w8139:bool)
        n4711 = Or(x="Tp1 normal speed gui", y="Tp1 auto normal speed") -> (x .or. y?=w8135:bool)
        n4712 = case shown="True" w8124 {
          tunnel: [FALSE w8151] -> w8121
          frame False {
          }
          frame True {
            n4713 = case shown="False" "tp1 start safety" {
              tunnel: [FALSE TRUE] -> w8151
              frame False {
                n4714 = local write "Warning Message"("CH1 TP cannot be started.\n" ("Error Message")) -> ()
                n4715 = local write "Tp1 auto start"(FALSE ("Tp1_auto_start")) -> ()
              }
              frame True {
              }
            }
          }
        }
        n4716 = Build Array(FALSE, w8121, w8126, w8141, w8139, w8135, "Tp1 Start initial", "Tp1 Stop initial") -> (w8147:bool[])
        n4717 = Boolean Array To Number(Boolean array=w8147) -> (number=w8148:u32)
        n4718 = Mantissa & Exponent(0:w8148) -> (2:w8146:dbl)  [unwired: 1 out]
        n4719 = case shown="3" w8146 {
          tunnel: w8123 -> [w8159 w8271 w8307 w8349 w8392 w8427 w8461 w8495]
          tunnel: w8122 -> [w8158 w8270 w8306 w8348 w8391 w8426 w8460 w8494]
          tunnel: [w8157 w8269 w8305 w8347 w8390 w8425 w8459 w8493] -> w8145